vi "CompleteLabView (3).vi"() -> ()   [LabVIEW 2022 SP3]
panel:
  out "Selected time":string
  in  "UYST":bool
  in  "HST":bool
  in  "AKST":bool
  in  "PST":bool
  in  "MST":bool
  in  "CST":bool
  in  "EST":bool
  in  "NZST":bool
  in  "AEDT":bool
  in  "PGT":bool
  in  "JST":bool
  in  "HKT":bool
  in  "THA":bool
  in  "BST":bool
  in  "PKT":bool
  in  "GST":bool
  in  "AST":bool
  in  "CAT":bool
  in  "CET":bool
  in  "UTC":bool
  in  "CVT":bool
  in  "ART":bool
  in  "AST":bool
  in  "Hawaii-Aleutian Time (HST)":bool
  in  "Alaska Standard Time (AKST)":bool
  in  "Pacific Zone Time (PT)":bool
  in  "Eastern Standard Time (EST)":bool
  in  "Central Standard Time (CST)":bool
  in  "Mountain Time (MST) 16":bool
  in  "New Zealand Standard Time":bool
  in  "Australian Eastern Time (AEDT)":bool
  in  "Papua New Guinea Time (PGT)":bool
  in  "Japan Standard Time":bool
  in  "Hong Kong Time (HKT)":bool
  in  "Thailand Standard Time (THA)":bool
  in  "Bangladesh Standard Time (BST)":bool
  in  "Pakistan Standard Time":bool
  in  "Gulf Standard Time (GST)":bool
  in  "Arabia Standard Time (AST)":bool
  in  "Central Africa Time (CAT)":bool
  in  "Central European Time (CET)":bool
  in  "Coordinated Universal Time (UTC)":bool
  in  "Cape Verde Time (CVT)":bool
  in  "Uruguay Summer Time":bool
  in  "Argentina Time":bool
  in  "Atlantic Standard Time (AST)":bool
  in  "stop":bool
  out "Current UTC Time":string
  # "Directions:\n Please click on the desired time zone. On-click the time will display, but when released show the base time. \n(Click the time zone on the map not below)"
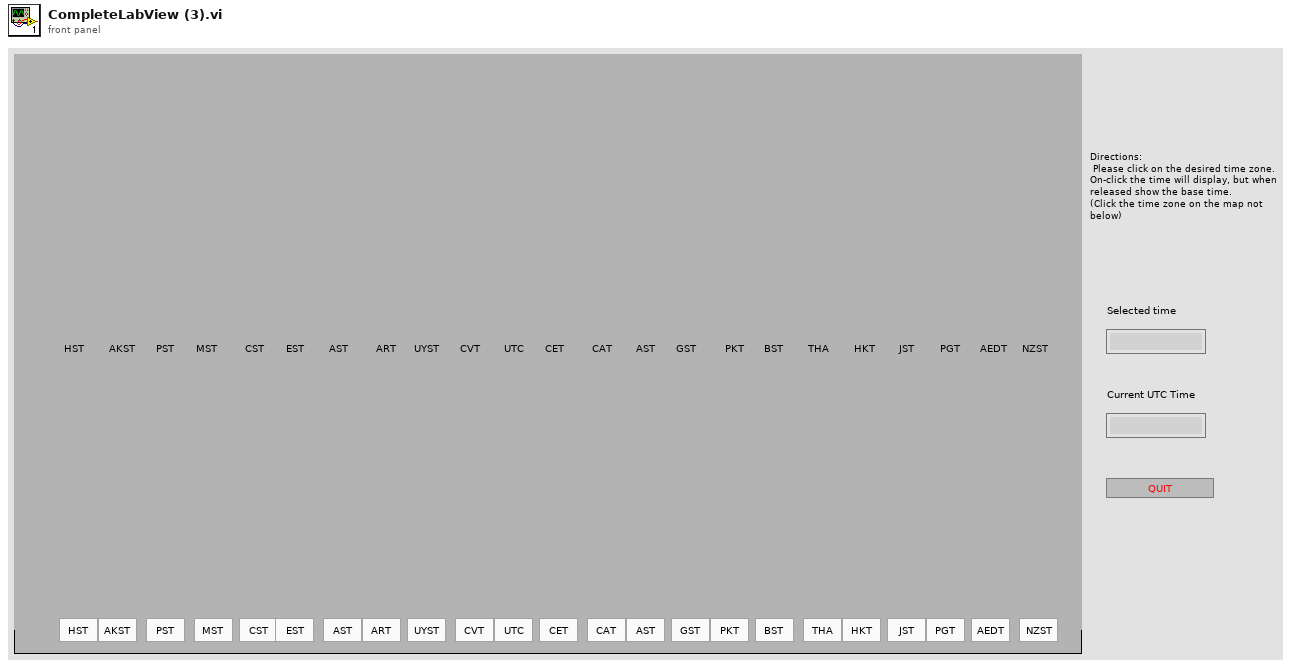
[diagram p1: front panel]
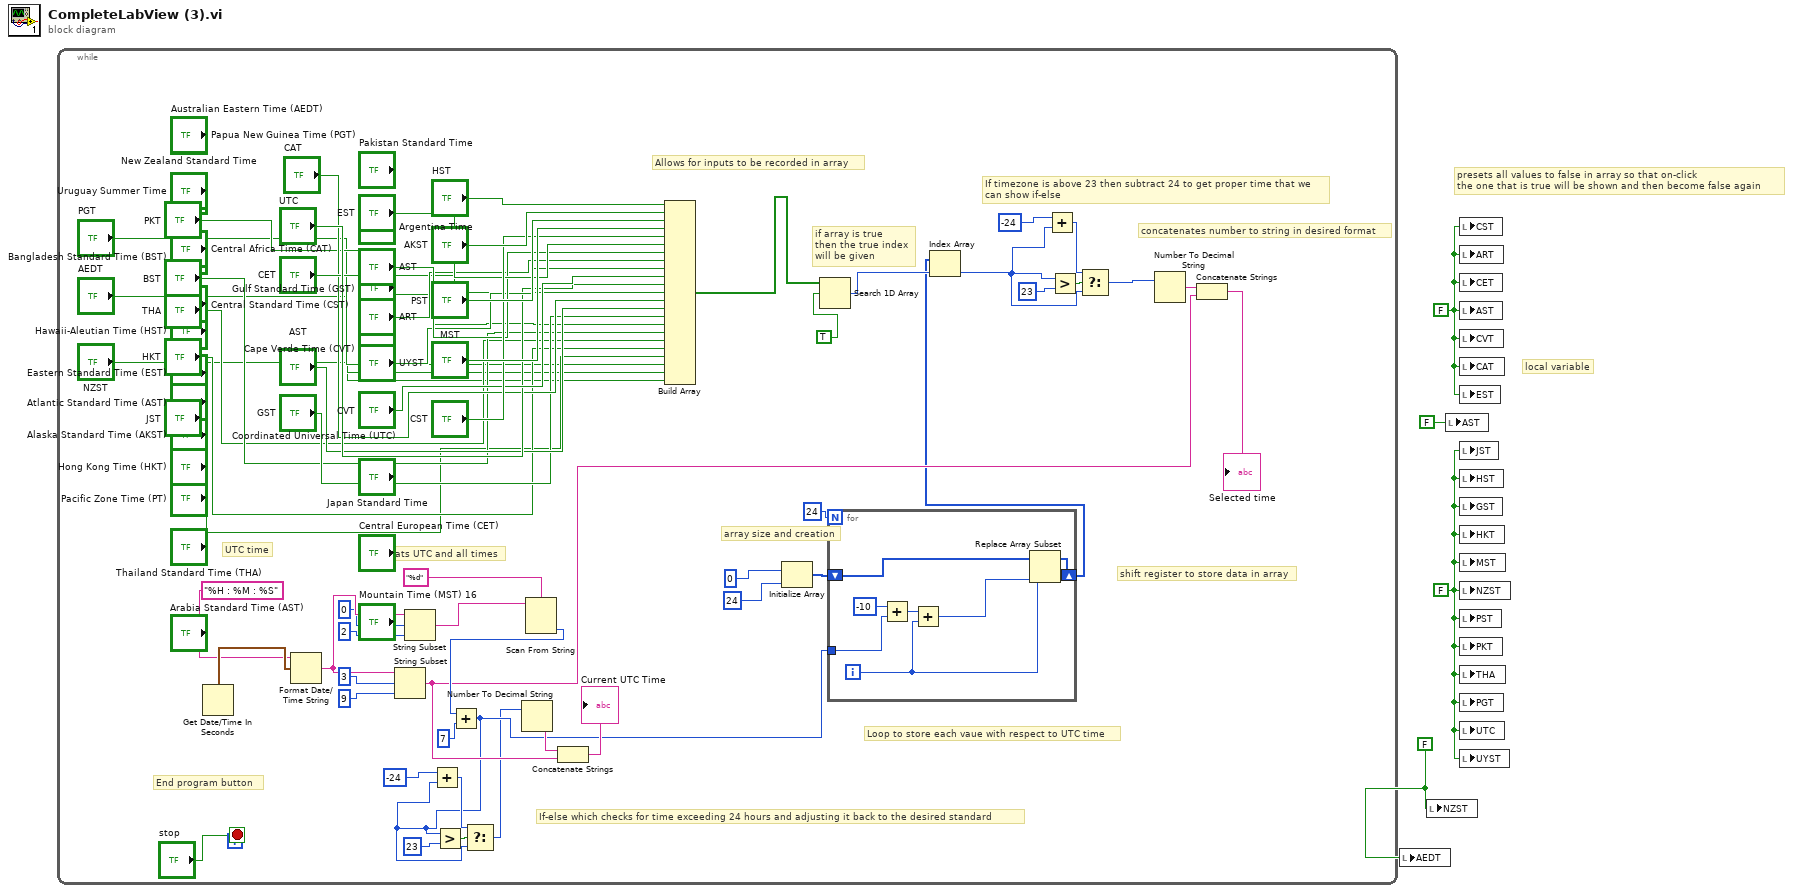
[diagram p0: block diagram]
diagram:
  w1 = FALSE
  w2 = FALSE
  w3 = FALSE
  # "local variable"
  # "presets all values to false in array so that on-click\nthe one that is true will be shown and then become false again"
  n1 = while {
    stop <- "stop" stop-if-true
    # "If-else which checks for time exceeding 24 hours and adjusting it back to the desired standard"
    # "formats UTC and all times"
    # "array size and creation"
    # "concatenates number to string in desired format"
    # "shift register to store data in array"
    # "If timezone is above 23 then subtract 24 to get proper time that we\ncan show if-else"
    # "Loop to store each vaue with respect to UTC time"
    # "End program button"
    # "UTC time"
    # "if array is true \nthen the true index\nwill be given"
    # "Allows for inputs to be recorded in array"
    n2 = Get Date/Time In Seconds() -> (seconds since 1Jan1904=w63:timestamp)
    n3 = Format Date/Time String(time format string (%c)="%H : %M : %S", seconds (now)=w63) -> (date/time string=w60:string)  [unwired: 1 in]
    n4 = String Subset(string=w60, offset (0)=3, length (rest)=9) -> (substring=w24:string)
    n5 = String Subset(string=w60, offset (0)=0, length (rest)=2) -> (substring=w62:string)
    n6 = Scan From String(format string="%d", input string=w62) -> (output 1=w61:i32)  [unwired: 3 in, 3 out]
    n7 = Add(x=w61, y=7) -> (x+y=w6:i32)
    n8 = Add(x=-24, y=w6) -> (x+y=w8:i32)
    n9 = Greater?(x=w6, y=23) -> (0:w9:bool)
    n10 = Select(t=w8, s=w9, f=w6) -> (s? t:f=w5:i32)
    n11 = Number To Decimal String(number=w5) -> (decimal integer string=w59:string)  [unwired: 1 in]
    n12 = Concatenate Strings(w59, w24) -> (→"Current UTC Time":string)
    n13 = Build Array("HST", "AKST", "PST", "MST", "CST", "EST", "AST", "ART", "UYST", "CVT", "UTC", "CET", "CAT", "AST", "GST", "PKT", "BST", "THA", "HKT", "JST", "PGT", "AEDT", "NZST") -> (w11:bool[])
    n14 = Initialize Array(0, 24) -> (w21:i32[])
    n15 = Search 1D Array(1D array=w11, element=TRUE) -> (index of element=w25:i32)  [unwired: 1 in]
    n16 = for {
      N: 24 -> [_]
      shift-right: [w66] -> w18
      shift-left: w21 -> [w68]
      tunnel: w6 -> [w70]
      i -> [w67]
      n17 = Add(x=-10, y=w70) -> (x+y=w69:i32)
      n18 = Add(x=w69, y=w67) -> (x+y=w65:i32)
      n19 = Replace Array Subset(array=w68, new element=w65, index=w67) -> (w66:i32[])
    }
    n20 = Index Array(array=w18, index=w25) -> (element=w15:i32)
    n21 = Add(x=-24, y=w15) -> (x+y=w14:i32)
    n22 = Greater?(x=w15, y=23) -> (0:w16:bool)
    n23 = Select(t=w14, s=w16, f=w15) -> (s? t:f=w13:i32)
    n24 = Number To Decimal String(number=w13) -> (decimal integer string=w23:string)  [unwired: 1 in]
    n25 = Concatenate Strings(w23, w24) -> (→"Selected time":string)
  }
  n26 = local write "AEDT"(w1) -> ()
  n27 = local write "NZST"(w1) -> ()
  n28 = local write "AST"(FALSE) -> ()
  n29 = local write "CST"(w3) -> ()
  n30 = local write "ART"(w3) -> ()
  n31 = local write "CET"(w3) -> ()
  n32 = local write "AST"(w3) -> ()
  n33 = local write "CVT"(w3) -> ()
  n34 = local write "CAT"(w3) -> ()
  n35 = local write "EST"(w3) -> ()
  n36 = local write "JST"(w2) -> ()
  n37 = local write "HST"(w2) -> ()
  n38 = local write "GST"(w2) -> ()
  n39 = local write "HKT"(w2) -> ()
  n40 = local write "MST"(w2) -> ()
  n41 = local write "NZST"(w2) -> ()
  n42 = local write "PST"(w2) -> ()
  n43 = local write "PKT"(w2) -> ()
  n44 = local write "THA"(w2) -> ()
  n45 = local write "PGT"(w2) -> ()
  n46 = local write "UTC"(w2) -> ()
  n47 = local write "UYST"(w2) -> ()
